vi "FlexMag - 23-03-2023.vi"() -> ()   [LabVIEW 2018] (continued)
    n13659 = local read "TRNS atm alg"() -> (w18628:bool)
    n13660 = Or(x=w18628, y=w18610) -> (x .or. y?=w18627:bool)
    n13661 = case shown="True" w18627 {
      tunnel: w18610 -> [_ w18926]
      frame False {
      }
      frame True {
        w18927 = FALSE ("TRNS atm alg")
        # "decision box"
        n13662 = local read "present location"() -> (w18952:dbl)
        n13663 = local read "target chamber"() -> (w18948:dbl)
        n13664 = Equal?(x=w18952, y=1.0) -> (x = y?=w18947:bool)
        n13665 = Equal?(x=w18952, y=2.0) -> (x = y?=w18946:bool)
        n13666 = Equal?(x=w18952, y=3.0) -> (x = y?=w18945:bool)
        n13667 = Equal?(x=w18952, y=4.0) -> (x = y?=w18944:bool)
        n13668 = Equal?(x=w18948, y=1.0) -> (x = y?=w18940:bool)
        n13669 = Equal?(x=w18948, y=2.0) -> (x = y?=w18941:bool)
        n13670 = Equal?(x=w18948, y=3.0) -> (x = y?=w18942:bool)
        n13671 = Equal?(x=w18948, y=4.0) -> (x = y?=w18943:bool)
        n13672 = local write "activate all trns sensors"(TRUE ("activate all trns sensors")) -> ()
        n13673 = And(x=w18947, y=w18940) -> ()  [unwired: 1 out]
        n13674 = And(x=w18947, y=w18941) -> (x .and. y?=→"1-2 tr":bool)
        n13675 = And(x=w18947, y=w18942) -> (x .and. y?=→"1-3 tr":bool)
        n13676 = And(x=w18947, y=w18943) -> (x .and. y?=→"1-4 tr":bool)
        n13677 = And(x=w18946, y=w18940) -> (x .and. y?=→"2-1 tr":bool)
        n13678 = And(x=w18946, y=w18941) -> ()  [unwired: 1 out]
        n13679 = And(x=w18946, y=w18942) -> (x .and. y?=→"2-3 tr":bool)
        n13680 = And(x=w18946, y=w18943) -> (x .and. y?=→"2-4 tr":bool)
        n13681 = local write "TRNS atm alg"(w18927) -> ()
        n13682 = local write "TRNS vacuum alg"(w18927) -> ()
        n13683 = And(x=w18945, y=w18940) -> (x .and. y?=→"3-1 tr":bool)
        n13684 = And(x=w18945, y=w18941) -> (x .and. y?=→"3-2 tr":bool)
        n13685 = And(x=w18945, y=w18942) -> ()  [unwired: 1 out]
        n13686 = And(x=w18945, y=w18943) -> (x .and. y?=→"3-4 tr":bool)
        n13687 = And(x=w18944, y=w18940) -> (x .and. y?=→"4-1 tr":bool)
        n13688 = And(x=w18944, y=w18941) -> (x .and. y?=→"4-2 tr":bool)
        n13689 = And(x=w18944, y=w18942) -> (x .and. y?=→"4-3 tr":bool)
        n13690 = And(x=w18944, y=w18943) -> ()  [unwired: 1 out]
        "trns V?" <- w18926
      }
    }
    n13691 = local read "1-2 tr"() -> (w18622:bool)
    n13692 = local read "1-3 tr"() -> (w18621:bool)
    n13693 = local read "1-4 tr"() -> (w18620:bool)
    n13694 = local read "2-1 tr"() -> (w18619:bool)
    n13695 = local read "2-3 tr"() -> (w18618:bool)
    n13696 = local read "2-4 tr"() -> (w18617:bool)
    n13697 = local read "3-1 tr"() -> (w18616:bool)
    n13698 = local read "3-2 tr"() -> (w18615:bool)
    n13699 = local read "3-4 tr"() -> (w18614:bool)
    n13700 = local read "4-1 tr"() -> (w18613:bool)
    n13701 = local read "4-2 tr"() -> (w18612:bool)
    n13702 = local read "4-3 tr"() -> (w18611:bool)
    n13703 = Build Array(FALSE, w18622, w18621, w18620, w18619, w18618, w18617, w18616, w18615, w18614, w18613, w18612, w18611) -> (w18625:bool[])
    n13704 = Boolean Array To Number(Boolean array=w18625) -> (number=w18626:u32)
    n13705 = Mantissa & Exponent(0:w18626) -> (2:w18623:dbl)  [unwired: 1 out]
    n13706 = case shown="12" w18623 {
      frame 0, Default {
      }
      frame 1 {
        # "1-2 tr"
        n13707 = stacked-sequence {
          frame #0 {
            n13708 = local read "trns error"() -> (w18643:bool)
            n13709 = local read "ABORT"() -> (w18642:bool)
            n13710 = Or(x=w18642, y=w18643) -> (x .or. y?=w18641:bool)
            n13711 = case shown="False" w18641 {
              frame False {
                n13712 = local write "ch1-2 transfer"(TRUE ("ch1-2 transfer")) -> ()
              }
              frame True {
              }
            }
          }
          frame #1 {
            n13713 = local read "trns error"() -> (w18647:bool)
            n13714 = local read "ABORT"() -> (w18646:bool)
            n13715 = Or(x=w18646, y=w18647) -> (x .or. y?=w18645:bool)
            n13716 = case shown="False" w18645 {
              frame False {
                n13717 = Wait (ms)(milliseconds to wait=u32 1000) -> ()  [unwired: 1 out]
              }
              frame True {
              }
            }
          }
          frame #2 {
            n13718 = while {
              stop <- w18649 stop-if-true
              n13719 = local read "ch1-2 transfer"() -> (w18653:bool)
              n13720 = local read "ABORT"() -> (w18652:bool)
              n13721 = Not(x=w18653) -> (.not. x?=w18651:bool)
              n13722 = Wait Until Next ms Multiple(millisecond multiple=u32 300) -> ()  [unwired: 1 out]
              n13723 = Compound Arithmetic op=OR(w18652, w18651) -> (w18649:bool)
            }
          }
          frame #3 {
            n13724 = local read "ABORT"() -> (w18654:bool)
            n13725 = case shown="False" w18654 {
              frame False {
                n13726 = local write "1-2 tr"(FALSE ("ch1-2 transfer")) -> ()
              }
              frame True {
              }
            }
          }
        }
      }
      frame 2 {
        # "1-3 tr"
        n13727 = stacked-sequence {
          frame #0 {
            n13728 = local read "trns error"() -> (w18656:bool)
            n13729 = local read "ABORT"() -> (w18657:bool)
            n13730 = Or(x=w18657, y=w18656) -> (x .or. y?=w18658:bool)
            n13731 = case shown="False" w18658 {
              frame False {
                n13732 = local write "ch1-2 transfer"(TRUE ("ch1-2 transfer")) -> ()
              }
              frame True {
              }
            }
          }
          frame #1 {
            n13733 = local read "trns error"() -> (w18662:bool)
            n13734 = local read "ABORT"() -> (w18661:bool)
            n13735 = Or(x=w18661, y=w18662) -> (x .or. y?=w18660:bool)
            n13736 = case shown="False" w18660 {
              frame False {
                n13737 = Wait (ms)(milliseconds to wait=u32 1000) -> ()  [unwired: 1 out]
              }
              frame True {
              }
            }
          }
          frame #2 {
            n13738 = while {
              stop <- w18664 stop-if-true
              n13739 = local read "ch1-2 transfer"() -> (w18668:bool)
              n13740 = local read "ABORT"() -> (w18667:bool)
              n13741 = Not(x=w18668) -> (.not. x?=w18666:bool)
              n13742 = Wait Until Next ms Multiple(millisecond multiple=u32 300) -> ()  [unwired: 1 out]
              n13743 = Compound Arithmetic op=OR(w18667, w18666) -> (w18664:bool)
            }
          }
          frame #3 {
            n13744 = local read "trns error"() -> (w18671:bool)
            n13745 = local read "ABORT"() -> (w18670:bool)
            n13746 = Or(x=w18670, y=w18671) -> (x .or. y?=w18669:bool)
            n13747 = case shown="False" w18669 {
              frame False {
                n13748 = local write "ch2-3 transfer"(TRUE ("ch2-3 transfer")) -> ()
              }
              frame True {
              }
            }
          }
          frame #4 {
            n13749 = local read "trns error"() -> (w18675:bool)
            n13750 = local read "ABORT"() -> (w18674:bool)
            n13751 = Or(x=w18674, y=w18675) -> (x .or. y?=w18673:bool)
            n13752 = case shown="False" w18673 {
              frame False {
                n13753 = Wait (ms)(milliseconds to wait=u32 1000) -> ()  [unwired: 1 out]
              }
              frame True {
              }
            }
          }
          frame #5 {
            n13754 = while {
              stop <- w18677 stop-if-true
              n13755 = Wait Until Next ms Multiple(millisecond multiple=u32 300) -> ()  [unwired: 1 out]
              n13756 = local read "ch2-3 transfer"() -> (w18681:bool)
              n13757 = local read "ABORT"() -> (w18680:bool)
              n13758 = Not(x=w18681) -> (.not. x?=w18679:bool)
              n13759 = Compound Arithmetic op=OR(w18680, w18679) -> (w18677:bool)
            }
          }
          frame #6 {
            n13760 = local read "ABORT"() -> (w18682:bool)
            n13761 = case shown="False" w18682 {
              frame False {
                n13762 = local write "1-3 tr"(FALSE ("1-3 tr")) -> ()
              }
              frame True {
              }
            }
          }
        }
      }
      frame 3 {
        # "1-4 tr"
        n13763 = stacked-sequence {
          frame #0 {
            n13764 = local read "trns error"() -> (w18686:bool)
            n13765 = local read "ABORT"() -> (w18685:bool)
            n13766 = Or(x=w18685, y=w18686) -> (x .or. y?=w18684:bool)
            n13767 = case shown="False" w18684 {
              frame False {
                n13768 = local write "ch1-2 transfer"(TRUE ("ch1-2 transfer")) -> ()
              }
              frame True {
              }
            }
          }
          frame #1 {
            n13769 = local read "ABORT"() -> (w18689:bool)
            n13770 = local read "trns error"() -> (w18690:bool)
            n13771 = Or(x=w18689, y=w18690) -> (x .or. y?=w18688:bool)
            n13772 = case shown="False" w18688 {
              frame False {
                n13773 = Wait (ms)(milliseconds to wait=u32 1000) -> ()  [unwired: 1 out]
              }
              frame True {
              }
            }
          }
          frame #2 {
            n13774 = while {
              stop <- w18692 stop-if-true
              n13775 = local read "ch1-2 transfer"() -> (w18696:bool)
              n13776 = local read "ABORT"() -> (w18695:bool)
              n13777 = Not(x=w18696) -> (.not. x?=w18694:bool)
              n13778 = Wait Until Next ms Multiple(millisecond multiple=u32 300) -> ()  [unwired: 1 out]
              n13779 = Compound Arithmetic op=OR(w18695, w18694) -> (w18692:bool)
            }
          }
          frame #3 {
            n13780 = local read "trns error"() -> (w18699:bool)
            n13781 = local read "ABORT"() -> (w18698:bool)
            n13782 = Or(x=w18698, y=w18699) -> (x .or. y?=w18697:bool)
            n13783 = case shown="False" w18697 {
              frame False {
                n13784 = local write "ch2-3 transfer"(TRUE ("ch2-3 transfer")) -> ()
              }
              frame True {
              }
            }
          }
          frame #4 {
            n13785 = local read "trns error"() -> (w18703:bool)
            n13786 = local read "ABORT"() -> (w18702:bool)
            n13787 = Or(x=w18702, y=w18703) -> (x .or. y?=w18701:bool)
            n13788 = case shown="False" w18701 {
              frame False {
                n13789 = Wait (ms)(milliseconds to wait=u32 1000) -> ()  [unwired: 1 out]
              }
              frame True {
              }
            }
          }
          frame #5 {
            n13790 = while {
              stop <- w18705 stop-if-true
              n13791 = Wait Until Next ms Multiple(millisecond multiple=u32 300) -> ()  [unwired: 1 out]
              n13792 = local read "ch2-3 transfer"() -> (w18709:bool)
              n13793 = local read "ABORT"() -> (w18708:bool)
              n13794 = Not(x=w18709) -> (.not. x?=w18707:bool)
              n13795 = Compound Arithmetic op=OR(w18708, w18707) -> (w18705:bool)
            }
          }
          frame #6 {
            n13796 = local read "trns error"() -> (w18712:bool)
            n13797 = local read "ABORT"() -> (w18711:bool)
            n13798 = Or(x=w18711, y=w18712) -> (x .or. y?=w18710:bool)
            n13799 = case shown="False" w18710 {
              frame False {
                n13800 = local write "ch3-4 transfer"(TRUE ("ch2-3 transfer")) -> ()
              }
              frame True {
              }
            }
          }
          frame #7 {
            n13801 = local read "ABORT"() -> (w18715:bool)
            n13802 = local read "trns error"() -> (w18716:bool)
            n13803 = Or(x=w18715, y=w18716) -> (x .or. y?=w18714:bool)
            n13804 = case shown="False" w18714 {
              frame False {
                n13805 = Wait (ms)(milliseconds to wait=u32 1000) -> ()  [unwired: 1 out]
              }
              frame True {
              }
            }
          }
          frame #8 {
            n13806 = while {
              stop <- w18718 stop-if-true
              n13807 = Wait Until Next ms Multiple(millisecond multiple=u32 300) -> ()  [unwired: 1 out]
              n13808 = local read "ch3-4 transfer"() -> (w18722:bool)
              n13809 = local read "ABORT"() -> (w18721:bool)
              n13810 = Not(x=w18722) -> (.not. x?=w18720:bool)
              n13811 = Compound Arithmetic op=OR(w18721, w18720) -> (w18718:bool)
            }
          }
          frame #9 {
            n13812 = local read "ABORT"() -> (w18723:bool)
            n13813 = case shown="False" w18723 {
              frame False {
                n13814 = local write "1-4 tr"(FALSE ("1-3 tr")) -> ()
              }
              frame True {
              }
            }
          }
        }
      }
      frame 4 {
        # "2-1 tr"
        n13815 = stacked-sequence {
          frame #0 {
            n13816 = local read "trns error"() -> (w18727:bool)
            n13817 = local read "ABORT"() -> (w18726:bool)
            n13818 = Or(x=w18726, y=w18727) -> (x .or. y?=w18725:bool)
            n13819 = case shown="False" w18725 {
              frame False {
                n13820 = local write "ch2-1 transfer"(TRUE ("ch1-2 transfer")) -> ()
              }
              frame True {
              }
            }
          }
          frame #1 {
            n13821 = local read "ABORT"() -> (w18730:bool)
            n13822 = local read "trns error"() -> (w18731:bool)
            n13823 = Or(x=w18730, y=w18731) -> (x .or. y?=w18729:bool)
            n13824 = case shown="False" w18729 {
              frame False {
                n13825 = Wait (ms)(milliseconds to wait=u32 1000) -> ()  [unwired: 1 out]
              }
              frame True {
              }
            }
          }
          frame #2 {
            n13826 = while {
              stop <- w18733 stop-if-true
              n13827 = local read "ch2-1 transfer"() -> (w18737:bool)
              n13828 = local read "ABORT"() -> (w18736:bool)
              n13829 = Not(x=w18737) -> (.not. x?=w18735:bool)
              n13830 = Wait Until Next ms Multiple(millisecond multiple=u32 300) -> ()  [unwired: 1 out]
              n13831 = Compound Arithmetic op=OR(w18736, w18735) -> (w18733:bool)
            }
          }
          frame #3 {
            n13832 = local read "ABORT"() -> (w18738:bool)
            n13833 = case shown="False" w18738 {
              frame False {
                n13834 = local write "2-1 tr"(FALSE ("1-3 tr")) -> ()
              }
              frame True {
              }
            }
          }
        }
      }
      frame 5 {
        # "2-3 tr"
        n13835 = stacked-sequence {
          frame #0 {
            n13836 = local read "ABORT"() -> (w18741:bool)
            n13837 = local read "trns error"() -> (w18742:bool)
            n13838 = Or(x=w18741, y=w18742) -> (x .or. y?=w18740:bool)
            n13839 = case shown="False" w18740 {
              frame False {
                n13840 = local write "ch2-3 transfer"(TRUE ("ch1-2 transfer")) -> ()
              }
              frame True {
              }
            }
          }
          frame #1 {
            n13841 = local read "trns error"() -> (w18746:bool)
            n13842 = local read "ABORT"() -> (w18745:bool)
            n13843 = Or(x=w18745, y=w18746) -> (x .or. y?=w18744:bool)
            n13844 = case shown="False" w18744 {
              frame False {
                n13845 = Wait (ms)(milliseconds to wait=u32 1000) -> ()  [unwired: 1 out]
              }
              frame True {
              }
            }
          }
          frame #2 {
            n13846 = while {
              stop <- w18748 stop-if-true
              n13847 = local read "ch2-3 transfer"() -> (w18752:bool)
              n13848 = local read "ABORT"() -> (w18751:bool)
              n13849 = Not(x=w18752) -> (.not. x?=w18750:bool)
              n13850 = Wait Until Next ms Multiple(millisecond multiple=u32 300) -> ()  [unwired: 1 out]
              n13851 = Compound Arithmetic op=OR(w18751, w18750) -> (w18748:bool)
            }
          }
          frame #3 {
            n13852 = local read "ABORT"() -> (w18753:bool)
            n13853 = case shown="False" w18753 {
              frame False {
                n13854 = local write "2-3 tr"(FALSE ("1-3 tr")) -> ()
              }
              frame True {
              }
            }
          }
        }
      }
      frame 6 {
        # "2-4 tr"
        n13855 = stacked-sequence {
          frame #0 {
            n13856 = local read "trns error"() -> (w18757:bool)
            n13857 = local read "ABORT"() -> (w18756:bool)
            n13858 = Or(x=w18756, y=w18757) -> (x .or. y?=w18755:bool)
            n13859 = case shown="False" w18755 {
              frame False {
                n13860 = local write "ch2-3 transfer"(TRUE ("ch1-2 transfer")) -> ()
              }
              frame True {
              }
            }
          }
          frame #1 {
            n13861 = local read "trns error"() -> (w18761:bool)
            n13862 = local read "ABORT"() -> (w18760:bool)
            n13863 = Or(x=w18760, y=w18761) -> (x .or. y?=w18759:bool)
            n13864 = case shown="False" w18759 {
              frame False {
                n13865 = Wait (ms)(milliseconds to wait=u32 1000) -> ()  [unwired: 1 out]
              }
              frame True {
              }
            }
          }
          frame #2 {
            n13866 = while {
              stop <- w18763 stop-if-true
              n13867 = local read "ch2-3 transfer"() -> (w18767:bool)
              n13868 = local read "ABORT"() -> (w18766:bool)
              n13869 = Not(x=w18767) -> (.not. x?=w18765:bool)
              n13870 = Wait Until Next ms Multiple(millisecond multiple=u32 300) -> ()  [unwired: 1 out]
              n13871 = Compound Arithmetic op=OR(w18766, w18765) -> (w18763:bool)
            }
          }
          frame #3 {
            n13872 = local read "trns error"() -> (w18770:bool)
            n13873 = local read "ABORT"() -> (w18769:bool)
            n13874 = Or(x=w18769, y=w18770) -> (x .or. y?=w18768:bool)
            n13875 = case shown="False" w18768 {
              frame False {
                n13876 = local write "ch3-4 transfer"(TRUE ("ch2-3 transfer")) -> ()
              }
              frame True {
              }
            }
          }
          frame #4 {
            n13877 = local read "trns error"() -> (w18774:bool)
            n13878 = local read "ABORT"() -> (w18773:bool)
            n13879 = Or(x=w18773, y=w18774) -> (x .or. y?=w18772:bool)
            n13880 = case shown="False" w18772 {
              frame False {
                n13881 = Wait (ms)(milliseconds to wait=u32 1000) -> ()  [unwired: 1 out]
              }
              frame True {
              }
            }
          }
          frame #5 {
            n13882 = while {
              stop <- w18776 stop-if-true
              n13883 = Wait Until Next ms Multiple(millisecond multiple=u32 300) -> ()  [unwired: 1 out]
              n13884 = local read "ch3-4 transfer"() -> (w18780:bool)
              n13885 = local read "ABORT"() -> (w18779:bool)
              n13886 = Not(x=w18780) -> (.not. x?=w18778:bool)
              n13887 = Compound Arithmetic op=OR(w18779, w18778) -> (w18776:bool)
            }
          }
          frame #6 {
            n13888 = local read "ABORT"() -> (w18781:bool)
            n13889 = case shown="False" w18781 {
              frame False {
                n13890 = local write "2-4 tr"(FALSE ("1-3 tr")) -> ()
              }
              frame True {
              }
            }
          }
        }
      }
      frame 7 {
        # "3-1 tr"
        n13891 = stacked-sequence {
          frame #0 {
            n13892 = local read "trns error"() -> (w18785:bool)
            n13893 = local read "ABORT"() -> (w18784:bool)
            n13894 = Or(x=w18784, y=w18785) -> (x .or. y?=w18783:bool)
            n13895 = case shown="False" w18783 {
              frame False {
                n13896 = local write "ch3-2 transfer"(TRUE ("ch1-2 transfer")) -> ()
              }
              frame True {
              }
            }
          }
          frame #1 {
            n13897 = local read "trns error"() -> (w18789:bool)
            n13898 = local read "ABORT"() -> (w18788:bool)
            n13899 = Or(x=w18788, y=w18789) -> (x .or. y?=w18787:bool)
            n13900 = case shown="False" w18787 {
              frame False {
                n13901 = Wait (ms)(milliseconds to wait=u32 1000) -> ()  [unwired: 1 out]
              }
              frame True {
              }
            }
          }
          frame #2 {
            n13902 = while {
              stop <- w18791 stop-if-true
              n13903 = local read "ch3-2 transfer"() -> (w18795:bool)
              n13904 = local read "ABORT"() -> (w18794:bool)
              n13905 = Not(x=w18795) -> (.not. x?=w18793:bool)
              n13906 = Wait Until Next ms Multiple(millisecond multiple=u32 300) -> ()  [unwired: 1 out]
              n13907 = Compound Arithmetic op=OR(w18794, w18793) -> (w18791:bool)
            }
          }
          frame #3 {
            n13908 = local read "trns error"() -> (w18798:bool)
            n13909 = local read "ABORT"() -> (w18797:bool)
            n13910 = Or(x=w18797, y=w18798) -> (x .or. y?=w18796:bool)
            n13911 = case shown="False" w18796 {
              frame False {
                n13912 = local write "ch2-1 transfer"(TRUE ("ch2-3 transfer")) -> ()
              }
              frame True {
              }
            }
          }
          frame #4 {
            n13913 = local read "trns error"() -> (w18802:bool)
            n13914 = local read "ABORT"() -> (w18801:bool)
            n13915 = Or(x=w18801, y=w18802) -> (x .or. y?=w18800:bool)
            n13916 = case shown="False" w18800 {
              frame False {
                n13917 = Wait (ms)(milliseconds to wait=u32 1000) -> ()  [unwired: 1 out]
              }
              frame True {
              }
            }
          }
          frame #5 {
            n13918 = while {
              stop <- w18804 stop-if-true
              n13919 = Wait Until Next ms Multiple(millisecond multiple=u32 300) -> ()  [unwired: 1 out]
              n13920 = local read "ch2-1 transfer"() -> (w18808:bool)
              n13921 = local read "ABORT"() -> (w18807:bool)
              n13922 = Not(x=w18808) -> (.not. x?=w18806:bool)
              n13923 = Compound Arithmetic op=OR(w18807, w18806) -> (w18804:bool)
            }
          }
          frame #6 {
            n13924 = local read "ABORT"() -> (w18809:bool)
            n13925 = case shown="False" w18809 {
              frame False {
                n13926 = local write "3-1 tr"(FALSE ("1-3 tr")) -> ()
              }
              frame True {
              }
            }
          }
        }
      }
      frame 8 {
        # "3-2 tr"
        n13927 = stacked-sequence {
          frame #0 {
            n13928 = local read "trns error"() -> (w18813:bool)
            n13929 = local read "ABORT"() -> (w18812:bool)
            n13930 = Or(x=w18812, y=w18813) -> (x .or. y?=w18811:bool)
            n13931 = case shown="False" w18811 {
              frame False {
                n13932 = local write "ch3-2 transfer"(TRUE ("ch1-2 transfer")) -> ()
              }
              frame True {
              }
            }
          }
          frame #1 {
            n13933 = local read "trns error"() -> (w18817:bool)
            n13934 = local read "ABORT"() -> (w18816:bool)
            n13935 = Or(x=w18816, y=w18817) -> (x .or. y?=w18815:bool)
            n13936 = case shown="False" w18815 {
              frame False {
                n13937 = Wait (ms)(milliseconds to wait=u32 1000) -> ()  [unwired: 1 out]
              }
              frame True {
              }
            }
          }
          frame #2 {
            n13938 = while {
              stop <- w18819 stop-if-true
              n13939 = local read "ch3-2 transfer"() -> (w18823:bool)
              n13940 = local read "ABORT"() -> (w18822:bool)
              n13941 = Not(x=w18823) -> (.not. x?=w18821:bool)
              n13942 = Wait Until Next ms Multiple(millisecond multiple=u32 300) -> ()  [unwired: 1 out]
              n13943 = Compound Arithmetic op=OR(w18822, w18821) -> (w18819:bool)
            }
          }
          frame #3 {
            n13944 = local read "ABORT"() -> (w18824:bool)
            n13945 = case shown="False" w18824 {
              frame False {
                n13946 = local write "3-2 tr"(FALSE ("1-3 tr")) -> ()
              }
              frame True {
              }
            }
          }
        }
      }
      frame 9 {
        # "3-4 tr"
        n13947 = stacked-sequence {
          frame #0 {
            n13948 = local read "trns error"() -> (w18828:bool)
            n13949 = local read "ABORT"() -> (w18827:bool)
            n13950 = Or(x=w18827, y=w18828) -> (x .or. y?=w18826:bool)
            n13951 = case shown="False" w18826 {
              frame False {
                n13952 = local write "ch3-4 transfer"(TRUE ("ch1-2 transfer")) -> ()
              }
              frame True {
              }
            }
          }
          frame #1 {
            n13953 = local read "trns error"() -> (w18832:bool)
            n13954 = local read "ABORT"() -> (w18831:bool)
            n13955 = Or(x=w18831, y=w18832) -> (x .or. y?=w18830:bool)
            n13956 = case shown="False" w18830 {
              frame False {
                n13957 = Wait (ms)(milliseconds to wait=u32 1000) -> ()  [unwired: 1 out]
              }
              frame True {
              }
            }
          }
          frame #2 {
            n13958 = while {
              stop <- w18834 stop-if-true
              n13959 = local read "ch3-4 transfer"() -> (w18838:bool)
              n13960 = local read "ABORT"() -> (w18837:bool)
              n13961 = Not(x=w18838) -> (.not. x?=w18836:bool)
              n13962 = Wait Until Next ms Multiple(millisecond multiple=u32 300) -> ()  [unwired: 1 out]
              n13963 = Compound Arithmetic op=OR(w18837, w18836) -> (w18834:bool)
            }
          }
          frame #3 {
            n13964 = local read "ABORT"() -> (w18839:bool)
            n13965 = case shown="False" w18839 {
              frame False {
                n13966 = local write "3-4 tr"(FALSE ("1-3 tr")) -> ()
              }
              frame True {
              }
            }
          }
        }
      }
      frame 10 {
        # "4-1 tr"
        n13967 = stacked-sequence {
          frame #0 {
            n13968 = local read "trns error"() -> (w18843:bool)
            n13969 = local read "ABORT"() -> (w18842:bool)
            n13970 = Or(x=w18842, y=w18843) -> (x .or. y?=w18841:bool)
            n13971 = case shown="False" w18841 {
              frame False {
                n13972 = local write "ch4-3 transfer"(TRUE ("ch1-2 transfer")) -> ()
              }
              frame True {
              }
            }
          }
          frame #1 {
            n13973 = local read "trns error"() -> (w18847:bool)
            n13974 = local read "ABORT"() -> (w18846:bool)
            n13975 = Or(x=w18846, y=w18847) -> (x .or. y?=w18845:bool)
            n13976 = case shown="False" w18845 {
              frame False {
                n13977 = Wait (ms)(milliseconds to wait=u32 1000) -> ()  [unwired: 1 out]
              }
              frame True {
              }
            }
          }
          frame #2 {
            n13978 = while {
              stop <- w18849 stop-if-true
              n13979 = local read "ch4-3 transfer"() -> (w18853:bool)
              n13980 = local read "ABORT"() -> (w18852:bool)
              n13981 = Not(x=w18853) -> (.not. x?=w18851:bool)
              n13982 = Wait Until Next ms Multiple(millisecond multiple=u32 300) -> ()  [unwired: 1 out]
              n13983 = Compound Arithmetic op=OR(w18852, w18851) -> (w18849:bool)
            }
          }
          frame #3 {
            n13984 = local read "trns error"() -> (w18856:bool)
            n13985 = local read "ABORT"() -> (w18855:bool)
            n13986 = Or(x=w18855, y=w18856) -> (x .or. y?=w18854:bool)
            n13987 = case shown="False" w18854 {
              frame False {
                n13988 = local write "ch3-2 transfer"(TRUE ("ch2-3 transfer")) -> ()
              }
              frame True {
              }
            }
          }
          frame #4 {
            n13989 = local read "trns error"() -> (w18860:bool)
            n13990 = local read "ABORT"() -> (w18859:bool)
            n13991 = Or(x=w18859, y=w18860) -> (x .or. y?=w18858:bool)
            n13992 = case shown="False" w18858 {
              frame False {
                n13993 = Wait (ms)(milliseconds to wait=u32 1000) -> ()  [unwired: 1 out]
              }
              frame True {
              }
            }
          }
          frame #5 {
            n13994 = while {
              stop <- w18862 stop-if-true
              n13995 = Wait Until Next ms Multiple(millisecond multiple=u32 300) -> ()  [unwired: 1 out]
              n13996 = local read "ch3-2 transfer"() -> (w18866:bool)
              n13997 = local read "ABORT"() -> (w18865:bool)
              n13998 = Not(x=w18866) -> (.not. x?=w18864:bool)
              n13999 = Compound Arithmetic op=OR(w18865, w18864) -> (w18862:bool)
            }
          }
          frame #6 {
            n14000 = local read "trns error"() -> (w18869:bool)
            n14001 = local read "ABORT"() -> (w18868:bool)
            n14002 = Or(x=w18868, y=w18869) -> (x .or. y?=w18867:bool)
            n14003 = case shown="False" w18867 {
              frame False {
                n14004 = local write "ch2-1 transfer"(TRUE ("ch2-3 transfer")) -> ()
              }
              frame True {
              }
            }
          }
          frame #7 {
            n14005 = local read "trns error"() -> (w18873:bool)
            n14006 = local read "ABORT"() -> (w18872:bool)
            n14007 = Or(x=w18872, y=w18873) -> (x .or. y?=w18871:bool)
            n14008 = case shown="False" w18871 {
              frame False {
                n14009 = Wait (ms)(milliseconds to wait=u32 1000) -> ()  [unwired: 1 out]
              }
              frame True {
              }
            }
          }
          frame #8 {
            n14010 = while {
              stop <- w18875 stop-if-true
              n14011 = Wait Until Next ms Multiple(millisecond multiple=u32 300) -> ()  [unwired: 1 out]
              n14012 = local read "ch2-1 transfer"() -> (w18879:bool)
              n14013 = local read "ABORT"() -> (w18878:bool)
              n14014 = Not(x=w18879) -> (.not. x?=w18877:bool)
              n14015 = Compound Arithmetic op=OR(w18878, w18877) -> (w18875:bool)
            }
          }
          frame #9 {
            n14016 = local read "ABORT"() -> (w18880:bool)
            n14017 = case shown="False" w18880 {
              frame False {
                n14018 = local write "4-1 tr"(FALSE ("1-3 tr")) -> ()
              }
              frame True {
              }
            }
          }
        }
      }
      frame 11 {
        # "4-2 tr"
        n14019 = stacked-sequence {
          frame #0 {
            n14020 = local read "trns error"() -> (w18884:bool)
            n14021 = local read "ABORT"() -> (w18883:bool)
            n14022 = Or(x=w18883, y=w18884) -> (x .or. y?=w18882:bool)
            n14023 = case shown="False" w18882 {
              frame False {
                n14024 = local write "ch4-3 transfer"(TRUE ("ch1-2 transfer")) -> ()
              }
              frame True {
              }
            }
          }
          frame #1 {
            n14025 = local read "trns error"() -> (w18888:bool)
            n14026 = local read "ABORT"() -> (w18887:bool)
            n14027 = Or(x=w18887, y=w18888) -> (x .or. y?=w18886:bool)
            n14028 = case shown="False" w18886 {
              frame False {
                n14029 = Wait (ms)(milliseconds to wait=u32 1000) -> ()  [unwired: 1 out]
              }
              frame True {
              }
            }
          }
          frame #2 {
            n14030 = while {
              stop <- w18890 stop-if-true
              n14031 = local read "ch4-3 transfer"() -> (w18894:bool)
              n14032 = local read "ABORT"() -> (w18893:bool)
              n14033 = Not(x=w18894) -> (.not. x?=w18892:bool)
              n14034 = Wait Until Next ms Multiple(millisecond multiple=u32 300) -> ()  [unwired: 1 out]
              n14035 = Compound Arithmetic op=OR(w18893, w18892) -> (w18890:bool)
            }
          }
          frame #3 {
            n14036 = local read "trns error"() -> (w18897:bool)
            n14037 = local read "ABORT"() -> (w18896:bool)
            n14038 = Or(x=w18896, y=w18897) -> (x .or. y?=w18895:bool)
            n14039 = case shown="False" w18895 {
              frame False {
                n14040 = local write "ch3-2 transfer"(TRUE ("ch2-3 transfer")) -> ()
              }
              frame True {
              }
            }
          }
          frame #4 {
            n14041 = local read "ABORT"() -> (w18900:bool)
            n14042 = local read "trns error"() -> (w18901:bool)
            n14043 = Or(x=w18900, y=w18901) -> (x .or. y?=w18899:bool)
            n14044 = case shown="False" w18899 {
              frame False {
                n14045 = Wait (ms)(milliseconds to wait=u32 1000) -> ()  [unwired: 1 out]
              }
              frame True {
              }
            }
          }
          frame #5 {
            n14046 = while {
              stop <- w18903 stop-if-true
              n14047 = Wait Until Next ms Multiple(millisecond multiple=u32 300) -> ()  [unwired: 1 out]
              n14048 = local read "ch3-2 transfer"() -> (w18907:bool)
              n14049 = local read "ABORT"() -> (w18906:bool)
              n14050 = Not(x=w18907) -> (.not. x?=w18905:bool)
              n14051 = Compound Arithmetic op=OR(w18906, w18905) -> (w18903:bool)
            }
          }
          frame #6 {
            n14052 = local read "ABORT"() -> (w18908:bool)
            n14053 = case shown="False" w18908 {
              frame False {
                n14054 = local write "4-2 tr"(FALSE ("1-3 tr")) -> ()
              }
              frame True {
              }
            }
          }
        }
      }
      frame 12 {
        # "4-3 tr"
        n14055 = stacked-sequence {
          frame #0 {
            n14056 = local read "trns error"() -> (w18912:bool)
            n14057 = local read "ABORT"() -> (w18911:bool)
            n14058 = Or(x=w18911, y=w18912) -> (x .or. y?=w18910:bool)
            n14059 = case shown="False" w18910 {
              frame False {
                n14060 = local write "ch4-3 transfer"(TRUE ("ch1-2 transfer")) -> ()
              }
              frame True {
              }
            }
          }
          frame #1 {
            n14061 = local read "trns error"() -> (w18916:bool)
            n14062 = local read "ABORT"() -> (w18915:bool)
            n14063 = Or(x=w18915, y=w18916) -> (x .or. y?=w18914:bool)
            n14064 = case shown="False" w18914 {
              frame False {
                n14065 = Wait (ms)(milliseconds to wait=u32 1000) -> ()  [unwired: 1 out]
              }
              frame True {
              }
            }
          }
          frame #2 {
            n14066 = while {
              stop <- w18918 stop-if-true
              n14067 = local read "ch4-3 transfer"() -> (w18922:bool)
              n14068 = local read "ABORT"() -> (w18921:bool)
              n14069 = Not(x=w18922) -> (.not. x?=w18920:bool)
              n14070 = Wait Until Next ms Multiple(millisecond multiple=u32 300) -> ()  [unwired: 1 out]
              n14071 = Compound Arithmetic op=OR(w18921, w18920) -> (w18918:bool)
            }
          }
          frame #3 {
            n14072 = local read "ABORT"() -> (w18923:bool)
            n14073 = case shown="False" w18923 {
              frame False {
                n14074 = local write "4-3 tr"(FALSE ("1-3 tr")) -> ()
              }
              frame True {
              }
            }
          }
        }
      }
    }
  }
  n14075 = while {
    stop <- FALSE stop-if-true
    n14076 = local read "abort ch1"() -> (w18980:bool)
    n14077 = local read "abort ch2"() -> (w18979:bool)
    n14078 = local read "abort ch3"() -> (w18978:bool)
    n14079 = local read "abort ch4"() -> (w18977:bool)
    n14080 = Wait Until Next ms Multiple(millisecond multiple=u32 300) -> ()  [unwired: 1 out]
    n14081 = Compound Arithmetic op=OR(w18980, w18979, w18978, w18977) -> (w18976:bool)
    n14082 = case shown="False" w18976 {
      frame False {
        n14083 = local read "ch1 pumpdown alg"() -> (w19065:bool)
        n14084 = local read "ch1 shutdown alg"() -> (w19026:bool)
        n14085 = local read "ch1 shutdown alg"() -> (w19025:bool)
        n14086 = local read "ch1 pumpdown alg"() -> (w19062:bool)
        n14087 = feedback #314() -> (w19063:bool)  [unwired: 1 in]
        n14088 = feedback-in #314("Pump Down CH1") -> ()
        n14089 = feedback #315() -> (w19018:bool)  [unwired: 1 in]
        n14090 = feedback-in #315("Shut Down CH1") -> ()
        n14091 = Implies(1:w19063, 2:"Pump Down CH1") -> (0:w19068:bool)
        n14092 = Implies(1:w19018, 2:"Shut Down CH1") -> (0:w19021:bool)
        n14093 = Implies(1:"Pump Down CH1", 2:w19063) -> (0:w19070:bool)
        n14094 = Implies(1:"Shut Down CH1", 2:w19018) -> (0:w19023:bool)
        n14095 = Not(x=w19068) -> (.not. x?=w19067:bool)
        n14096 = Not(x=w19021) -> (.not. x?=w19020:bool)
        n14097 = Not(x=w19070) -> (.not. x?=w19066:bool)
        n14098 = Not(x=w19065) -> (.not. x?=w19069:bool)
        n14099 = Not(x=w19023) -> (.not. x?=w19019:bool)
        n14100 = Not(x=w19026) -> (.not. x?=w19022:bool)
        n14101 = Compound Arithmetic op=AND(w19066, w19062) -> (w19060:bool)
        n14102 = Compound Arithmetic op=AND(w19069, w19067) -> (w19061:bool)
        n14103 = Compound Arithmetic op=AND(w19019, w19025) -> (w19016:bool)
        n14104 = Compound Arithmetic op=AND(w19022, w19020) -> (w19017:bool)
        n14105 = case shown="True" w19061 {
          frame False {
          }
          frame True {
            n14106 = stacked-sequence {
              frame #0 {
                n14107 = Two Button Dialog(message="Continue Chamber 1 Pump Down Process ?", 1:"No, Cancel" ("F button name (\"Cancel\")"), 2:"Yes, Continue" ("T button name (\"OK\")")) -> (T button?=→"ch1 pd continue":bool)
              }
              frame #1 {
                n14108 = Wait (ms)(milliseconds to wait=u32 100) -> ()  [unwired: 1 out]
              }
              frame #2 {
                n14109 = local read "ch1 pd continue"() -> (w19242:bool)
                n14110 = Wait (ms)(milliseconds to wait=u32 100) -> ()  [unwired: 1 out]
                n14111 = case shown="False" w19242 {
                  frame False {
                    w19243 = FALSE ("ch1 pumpdown alg")
                    n14112 = local write "ch1 pumpdown alg"(w19243) -> ()
                    n14113 = local write "Pump Down CH1"(w19243) -> ()
                  }
                  frame True {
                    n14114 = local write "ch1 pumpdown alg"(TRUE ("ch1 pumpdown alg")) -> ()
                  }
                }
              }
              frame #3 {
                n14115 = Wait (ms)(milliseconds to wait=u32 100) -> ()  [unwired: 1 out]
              }
              frame #4 {
                n14116 = local write "ch1 pd continue"(FALSE ("ch1 pd continue")) -> ()
              }
            }
          }
        }
        n14117 = case shown="True" w19060 {
          frame False {
          }
          frame True {
            n14118 = stacked-sequence {
              frame #0 {
                n14119 = Two Button Dialog(message="Cancel Chamber 1 Pump Down Process ?", 1:"No, Contunie" ("F button name (\"Cancel\")"), 2:"Yes, Cancel" ("T button name (\"OK\")")) -> (T button?=→"ch1 pd cancel":bool)
              }
              frame #1 {
                n14120 = Wait (ms)(milliseconds to wait=u32 100) -> ()  [unwired: 1 out]
              }
              frame #2 {
                n14121 = local read "ch1 pd cancel"() -> (w19231:bool)
                n14122 = Wait (ms)(milliseconds to wait=u32 100) -> ()  [unwired: 1 out]
                n14123 = case shown="False" w19231 {
                  frame False {
                    w19232 = TRUE ("ch1 pumpdown alg")
                    n14124 = local write "ch1 pumpdown alg"(w19232) -> ()
                    n14125 = local write "Pump Down CH1"(w19232) -> ()
                  }
                  frame True {
                    w19233 = FALSE ("ch1 pumpdown alg")
                    n14126 = local write "ch1 pumpdown alg"(w19233) -> ()
                    n14127 = local write "Pump Down CH1"(w19233) -> ()
                  }
                }
              }
              frame #3 {
                n14128 = Wait (ms)(milliseconds to wait=u32 100) -> ()  [unwired: 1 out]
              }
              frame #4 {
                n14129 = local write "ch1 pd cancel"(FALSE ("ch1 pd continue")) -> ()
              }
            }
          }
        }
        n14130 = case shown="True" w19017 {
          frame False {
          }
          frame True {
            n14131 = stacked-sequence {
              frame #0 {
                n14132 = Two Button Dialog(message="Continue Chamber 1 Shut Down Process ?", 1:"No, Cancel" ("F button name (\"Cancel\")"), 2:"Yes, Continue" ("T button name (\"OK\")")) -> (T button?=→"ch1 sd continue":bool)
              }
              frame #1 {
                n14133 = Wait (ms)(milliseconds to wait=u32 100) -> ()  [unwired: 1 out]
              }
              frame #2 {
                n14134 = local read "ch1 sd continue"() -> (w19154:bool)
                n14135 = Wait (ms)(milliseconds to wait=u32 100) -> ()  [unwired: 1 out]
                n14136 = case shown="False" w19154 {
                  frame False {
                    w19155 = FALSE ("ch1 pumpdown alg")
                    n14137 = local write "ch1 shutdown alg"(w19155) -> ()
                    n14138 = local write "Shut Down CH1"(w19155) -> ()
                  }
                  frame True {
                    n14139 = local write "ch1 shutdown alg"(TRUE ("ch1 pumpdown alg")) -> ()
                  }
                }
              }
              frame #3 {
                n14140 = Wait (ms)(milliseconds to wait=u32 100) -> ()  [unwired: 1 out]
              }
              frame #4 {
                n14141 = local write "ch1 sd continue"(FALSE ("ch1 pd continue")) -> ()
              }
            }
          }
        }
        n14142 = case shown="True" w19016 {
          frame False {
          }
          frame True {
            n14143 = stacked-sequence {
              frame #0 {
                n14144 = Two Button Dialog(message="Cancel Chamber 1 Shut Down Process ?", 1:"No, Contunie" ("F button name (\"Cancel\")"), 2:"Yes, Cancel" ("T button name (\"OK\")")) -> (T button?=→"ch1 sd cancel":bool)
              }
              frame #1 {
                n14145 = Wait (ms)(milliseconds to wait=u32 100) -> ()  [unwired: 1 out]
              }
              frame #2 {
                n14146 = local read "ch1 sd cancel"() -> (w19143:bool)
                n14147 = Wait (ms)(milliseconds to wait=u32 100) -> ()  [unwired: 1 out]
                n14148 = case shown="True" w19143 {
                  frame False {
                    w19144 = TRUE ("ch1 pumpdown alg")
                    n14149 = local write "ch1 shutdown alg"(w19144) -> ()
                    n14150 = local write "Shut Down CH1"(w19144) -> ()
                  }
                  frame True {
                    w19145 = FALSE ("ch1 pumpdown alg")
                    n14151 = local write "ch1 shutdown alg"(w19145) -> ()
                    n14152 = local write "Shut Down CH1"(w19145) -> ()
                  }
                }
              }
              frame #3 {
                n14153 = Wait (ms)(milliseconds to wait=u32 100) -> ()  [unwired: 1 out]
              }
              frame #4 {
                n14154 = local write "ch1 sd cancel"(FALSE ("ch1 pd continue")) -> ()
              }
            }
          }
        }
        n14155 = local read "ch2 pumpdown alg"() -> (w19049:bool)
        n14156 = local read "ch2 pumpdown alg"() -> (w19050:bool)
        n14157 = local read "ch2 shutdown alg"() -> (w19005:bool)
        n14158 = local read "ch2 shutdown alg"() -> (w19006:bool)
        n14159 = feedback #316() -> (w19057:bool)  [unwired: 1 in]
        n14160 = feedback-in #316("Pump Down CH2") -> ()
        n14161 = feedback #317() -> (w19013:bool)  [unwired: 1 in]
        n14162 = feedback-in #317("Shut Down CH2") -> ()
        n14163 = Implies(1:w19057, 2:"Pump Down CH2") -> (0:w19054:bool)
        n14164 = Implies(1:w19013, 2:"Shut Down CH2") -> (0:w19010:bool)
        n14165 = Implies(1:"Pump Down CH2", 2:w19057) -> (0:w19052:bool)
        n14166 = Implies(1:"Shut Down CH2", 2:w19013) -> (0:w19008:bool)
        n14167 = Not(x=w19054) -> (.not. x?=w19055:bool)
        n14168 = Not(x=w19010) -> (.not. x?=w19011:bool)
        n14169 = Not(x=w19052) -> (.not. x?=w19056:bool)
        n14170 = Not(x=w19049) -> (.not. x?=w19053:bool)
        n14171 = Not(x=w19008) -> (.not. x?=w19012:bool)
        n14172 = Not(x=w19005) -> (.not. x?=w19009:bool)
        n14173 = Compound Arithmetic op=AND(w19056, w19050) -> (w19059:bool)
        n14174 = Compound Arithmetic op=AND(w19053, w19055) -> (w19058:bool)
        n14175 = Compound Arithmetic op=AND(w19012, w19006) -> (w19015:bool)
        n14176 = Compound Arithmetic op=AND(w19009, w19011) -> (w19014:bool)
        n14177 = case shown="True" w19058 {
          frame False {
          }
          frame True {
            n14178 = stacked-sequence {
              frame #0 {
                n14179 = Two Button Dialog(message="Continue Chamber 2 Pump Down Process ?", 1:"No, Cancel" ("F button name (\"Cancel\")"), 2:"Yes, Continue" ("T button name (\"OK\")")) -> (T button?=→"ch2 pd continue":bool)
              }
              frame #1 {
                n14180 = Wait (ms)(milliseconds to wait=u32 100) -> ()  [unwired: 1 out]
              }
              frame #2 {
                n14181 = local read "ch2 pd continue"() -> (w19220:bool)
                n14182 = Wait (ms)(milliseconds to wait=u32 100) -> ()  [unwired: 1 out]
                n14183 = case shown="False" w19220 {
                  frame False {
                    w19221 = FALSE ("ch1 pumpdown alg")
                    n14184 = local write "ch2 pumpdown alg"(w19221) -> ()
                    n14185 = local write "Pump Down CH2"(w19221) -> ()
                  }
                  frame True {
                    n14186 = local write "ch2 pumpdown alg"(TRUE ("ch1 pumpdown alg")) -> ()
                  }
                }
              }
              frame #3 {
                n14187 = Wait (ms)(milliseconds to wait=u32 100) -> ()  [unwired: 1 out]
              }
              frame #4 {
                n14188 = local write "ch2 pd continue"(FALSE ("ch1 pd continue")) -> ()
              }
            }
          }
        }
        n14189 = case shown="True" w19059 {
          frame False {
          }
          frame True {
            n14190 = stacked-sequence {
              frame #0 {
                n14191 = Two Button Dialog(message="Cancel Chamber 2 Pump Down Process ?", 1:"No, Contunie" ("F button name (\"Cancel\")"), 2:"Yes, Cancel" ("T button name (\"OK\")")) -> (T button?=→"ch2 pd cancel":bool)
              }
              frame #1 {
                n14192 = Wait (ms)(milliseconds to wait=u32 100) -> ()  [unwired: 1 out]
              }
              frame #2 {
                n14193 = local read "ch2 pd cancel"() -> (w19209:bool)
                n14194 = Wait (ms)(milliseconds to wait=u32 100) -> ()  [unwired: 1 out]
                n14195 = case shown="True" w19209 {
                  frame False {
                    w19210 = TRUE ("ch1 pumpdown alg")
                    n14196 = local write "ch2 pumpdown alg"(w19210) -> ()
                    n14197 = local write "Pump Down CH2"(w19210) -> ()
                  }
                  frame True {
                    w19211 = FALSE ("ch1 pumpdown alg")
                    n14198 = local write "ch2 pumpdown alg"(w19211) -> ()
                    n14199 = local write "Pump Down CH2"(w19211) -> ()
                  }
                }
              }
              frame #3 {
                n14200 = Wait (ms)(milliseconds to wait=u32 100) -> ()  [unwired: 1 out]
              }
              frame #4 {
                n14201 = local write "ch2 pd cancel"(FALSE ("ch1 pd continue")) -> ()
              }
            }
          }
        }
        n14202 = case shown="True" w19014 {
          frame False {
          }
          frame True {
            n14203 = stacked-sequence {
              frame #0 {
                n14204 = Two Button Dialog(message="Continue Chamber 2 Shut Down Process ?", 1:"No, Cancel" ("F button name (\"Cancel\")"), 2:"Yes, Continue" ("T button name (\"OK\")")) -> (T button?=→"ch2 sd continue":bool)
              }
              frame #1 {
                n14205 = Wait (ms)(milliseconds to wait=u32 100) -> ()  [unwired: 1 out]
              }
              frame #2 {
                n14206 = local read "ch2 sd continue"() -> (w19132:bool)
                n14207 = Wait (ms)(milliseconds to wait=u32 100) -> ()  [unwired: 1 out]
                n14208 = case shown="False" w19132 {
                  frame False {
                    w19133 = FALSE ("ch1 pumpdown alg")
                    n14209 = local write "ch2 shutdown alg"(w19133) -> ()
                    n14210 = local write "Shut Down CH2"(w19133) -> ()
                  }
                  frame True {
                    n14211 = local write "ch2 shutdown alg"(TRUE ("ch1 pumpdown alg")) -> ()
                  }
                }
              }
              frame #3 {
                n14212 = Wait (ms)(milliseconds to wait=u32 100) -> ()  [unwired: 1 out]
              }
              frame #4 {
                n14213 = local write "ch2 sd continue"(FALSE ("ch1 pd continue")) -> ()
              }
            }
          }
        }
        n14214 = case shown="True" w19015 {
          frame False {
          }
          frame True {
            n14215 = stacked-sequence {
              frame #0 {
                n14216 = Two Button Dialog(message="Cancel Chamber 2 Shut Down Process ?", 1:"No, Contunie" ("F button name (\"Cancel\")"), 2:"Yes, Cancel" ("T button name (\"OK\")")) -> (T button?=→"ch2 sd cancel":bool)
              }
              frame #1 {
                n14217 = Wait (ms)(milliseconds to wait=u32 100) -> ()  [unwired: 1 out]
              }
              frame #2 {
                n14218 = local read "ch2 sd cancel"() -> (w19121:bool)
                n14219 = Wait (ms)(milliseconds to wait=u32 100) -> ()  [unwired: 1 out]
                n14220 = case shown="False" w19121 {
                  frame False {
                    w19122 = TRUE ("ch1 pumpdown alg")
                    n14221 = local write "ch2 shutdown alg"(w19122) -> ()
                    n14222 = local write "Shut Down CH2"(w19122) -> ()
                  }
                  frame True {
                    w19123 = FALSE ("ch1 pumpdown alg")
                    n14223 = local write "ch2 shutdown alg"(w19123) -> ()
                    n14224 = local write "Shut Down CH2"(w19123) -> ()
                  }
                }
              }
              frame #3 {
                n14225 = Wait (ms)(milliseconds to wait=u32 100) -> ()  [unwired: 1 out]
              }
              frame #4 {
                n14226 = local write "ch2 sd cancel"(FALSE ("ch1 pd continue")) -> ()
              }
            }
          }
        }
        n14227 = local read "ch3 pumpdown alg"() -> (w19039:bool)
        n14228 = local read "ch3 pumpdown alg"() -> (w19040:bool)
        n14229 = local read "ch3 shutdown alg"() -> (w19004:bool)
        n14230 = local read "ch3 shutdown alg"() -> (w19003:bool)
        n14231 = feedback #318() -> (w19043:bool)  [unwired: 1 in]
        n14232 = feedback-in #318("Pump Down CH3") -> ()
        n14233 = feedback #319() -> (w18996:bool)  [unwired: 1 in]
        n14234 = feedback-in #319("Shut Down CH3") -> ()
        n14235 = Implies(1:w19043, 2:"Pump Down CH3") -> (0:w19046:bool)
        n14236 = Implies(1:w18996, 2:"Shut Down CH3") -> (0:w18999:bool)
        n14237 = Implies(1:"Pump Down CH3", 2:w19043) -> (0:w19048:bool)
        n14238 = Implies(1:"Shut Down CH3", 2:w18996) -> (0:w19001:bool)
        n14239 = Not(x=w19046) -> (.not. x?=w19045:bool)
        n14240 = Not(x=w18999) -> (.not. x?=w18998:bool)
        n14241 = Not(x=w19048) -> (.not. x?=w19044:bool)
        n14242 = Not(x=w19039) -> (.not. x?=w19047:bool)
        n14243 = Not(x=w19001) -> (.not. x?=w18997:bool)
        n14244 = Not(x=w19004) -> (.not. x?=w19000:bool)
        n14245 = Compound Arithmetic op=AND(w19044, w19040) -> (w19041:bool)
        n14246 = Compound Arithmetic op=AND(w19047, w19045) -> (w19042:bool)
        n14247 = Compound Arithmetic op=AND(w18997, w19003) -> (w18994:bool)
        n14248 = Compound Arithmetic op=AND(w19000, w18998) -> (w18995:bool)
        n14249 = case shown="True" w19042 {
          frame False {
          }
          frame True {
            n14250 = stacked-sequence {
              frame #0 {
                n14251 = Two Button Dialog(message="Continue Chamber 3 Pump Down Process ?", 1:"No, Cancel" ("F button name (\"Cancel\")"), 2:"Yes, Continue" ("T button name (\"OK\")")) -> (T button?=→"ch3 pd continue":bool)
              }
              frame #1 {
                n14252 = Wait (ms)(milliseconds to wait=u32 100) -> ()  [unwired: 1 out]
              }
              frame #2 {
                n14253 = local read "ch3 pd continue"() -> (w19198:bool)
                n14254 = Wait (ms)(milliseconds to wait=u32 100) -> ()  [unwired: 1 out]
                n14255 = case shown="True" w19198 {
                  frame False {
                    w19199 = FALSE ("ch1 pumpdown alg")
                    n14256 = local write "ch3 pumpdown alg"(w19199) -> ()
                    n14257 = local write "Pump Down CH3"(w19199) -> ()
                  }
                  frame True {
                    n14258 = local write "ch3 pumpdown alg"(TRUE ("ch1 pumpdown alg")) -> ()
                  }
                }
              }
              frame #3 {
                n14259 = Wait (ms)(milliseconds to wait=u32 100) -> ()  [unwired: 1 out]
              }
              frame #4 {
                n14260 = local write "ch3 pd continue"(FALSE ("ch1 pd continue")) -> ()
              }
            }
          }
        }
        n14261 = case shown="True" w19041 {
          frame False {
          }
          frame True {
            n14262 = stacked-sequence {
              frame #0 {
                n14263 = Two Button Dialog(message="Cancel Chamber 3 Pump Down Process ?", 1:"No, Contunie" ("F button name (\"Cancel\")"), 2:"Yes, Cancel" ("T button name (\"OK\")")) -> (T button?=→"ch3 pd cancel":bool)
              }
              frame #1 {
                n14264 = Wait (ms)(milliseconds to wait=u32 100) -> ()  [unwired: 1 out]
              }
              frame #2 {
                n14265 = local read "ch3 pd cancel"() -> (w19187:bool)
                n14266 = Wait (ms)(milliseconds to wait=u32 100) -> ()  [unwired: 1 out]
                n14267 = case shown="False" w19187 {
                  frame False {
                    w19188 = TRUE ("ch1 pumpdown alg")
                    n14268 = local write "ch3 pumpdown alg"(w19188) -> ()
                    n14269 = local write "Pump Down CH3"(w19188) -> ()
                  }
                  frame True {
                    w19189 = FALSE ("ch1 pumpdown alg")
                    n14270 = local write "ch3 pumpdown alg"(w19189) -> ()
                    n14271 = local write "Pump Down CH3"(w19189) -> ()
                  }
                }
              }
              frame #3 {
                n14272 = Wait (ms)(milliseconds to wait=u32 100) -> ()  [unwired: 1 out]
              }
              frame #4 {
                n14273 = local write "ch3 pd cancel"(FALSE ("ch1 pd continue")) -> ()
              }
            }
          }
        }
        n14274 = case shown="True" w18995 {
          frame False {